vi "drawRoi.vi"(6 "Colors (Red)":u32[](array[colorbox])=[16711680], 8 "bit depth":enum16{"16bits", "14bits", "12bits", "8bits"}(ring)=enum."12bits", 9 "ROI":refnum<vi>, 10 "Reff image":T1=refnum, 11 "Whole image":T1=refnum) -> (0 "size":i32=712674, 1 "mean":dbl=2650.364090734333, 2 "Reff image":T1(plugin-control), 3 "Image Out":T1, 4 "Percentile alert":bool)   [LabVIEW 2023]
uses:
  <vilib>/vision/Image Controls.llb/IMAQ Image.ctl
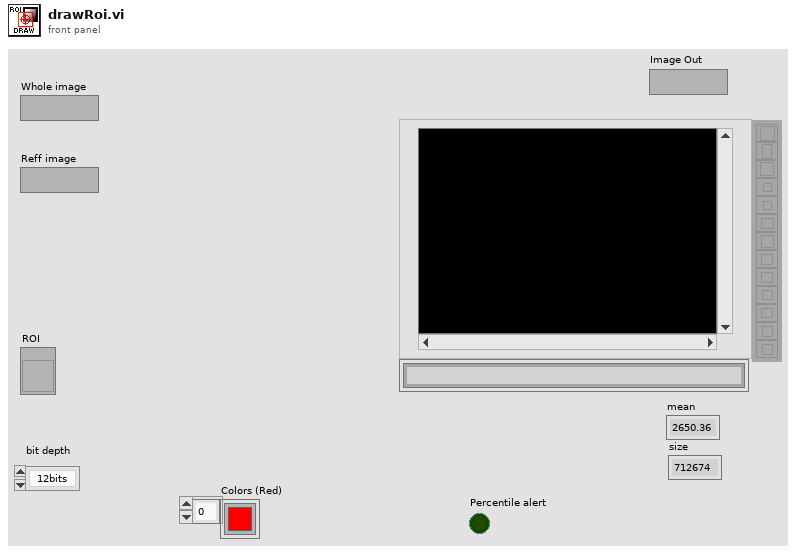
[diagram p1: front panel]
types:
  T1 = typedef "IMAQ Image.ctl" = refnum<image>
  T2 = cluster{"Global Rectangle":i32[], "Contours":cluster{"Contour Type":u32, "ROI Type":u32, "Points":i32[]}[]}
  T3 = cluster{"mean (ROI)":dbl, "max (ROI)":i16, "max_counts":dbl, "image_size":i32, "# Sat. Pixels":sgl, "# in percentile":dbl}
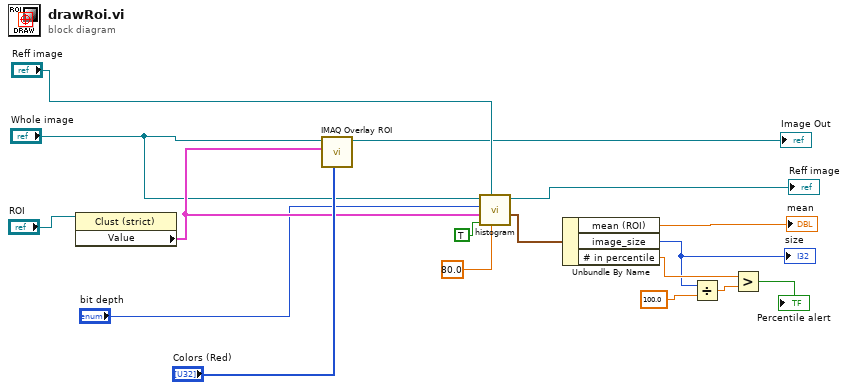
[diagram p0: block diagram]
diagram:
  n1 = property class="Clust (strict)"(reference="ROI") -> ("Value"=w15:T2)  [unwired: 1 in, 2 out]
  n2 = call "IMAQ Overlay ROI"("Colors (Green)"="Colors (Red)", "ROI Descriptor"=w15, "Image"="Whole image") -> ("Image Out"=→"Image Out":T1)  [unwired: 7 in, 1 out]
  n3 = call "histogram.vi"("Percentile check"=80.0, "Image ROI"="Reff image", "useROI"=TRUE, "ROI Descriptor"=w15, "bit depth"="bit depth", "Image"="Whole image") -> ("Statistics"=w10:T3, "Image Out (ROI)"=→"Reff image":T1)  [unwired: 1 in, 3 out]
  n4 = Unbundle By Name(w10) -> ("mean (ROI)"=→"mean":dbl, "image_size"=w3:i32, "# in percentile"=w5:dbl)
  "size" <- w3
  n5 = Divide(x=w3, y=100.0 ("Percentile check")) -> (x/y=w4:dbl)
  n6 = Greater?(x=w5, y=w4) -> (0:→"Percentile alert":bool)
